vi "Test UI.vi"() -> ()   [LabVIEW 2012]
uses:
  Controls/Settings.ctl
  Controls/Stop.ctl
  Controls/Altitude Xctl/Altitude2.xctl
panel:
  out "Altitude2":cluster{"time":timestamp, "altitude":dbl}(xcontrol)
  in  "Stop":T1
  in  "settings":T2
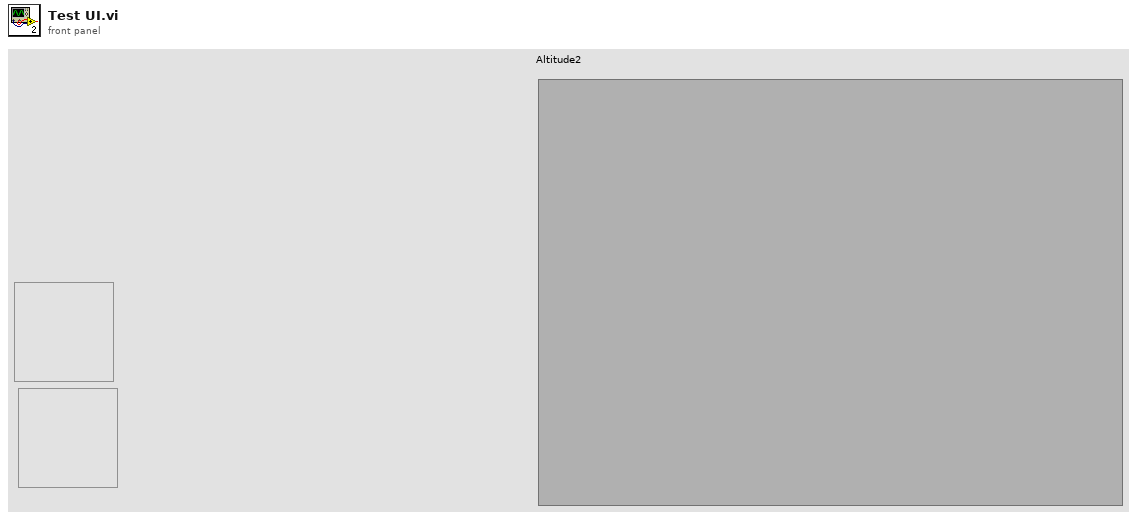
[diagram p1: front panel]
types:
  T1 = typedef "Stop.ctl" = bool
  T2 = typedef "Settings.ctl" = bool
  T3 = cluster{"seconds since 1Jan1904":timestamp, "number: 0 to 1":dbl}
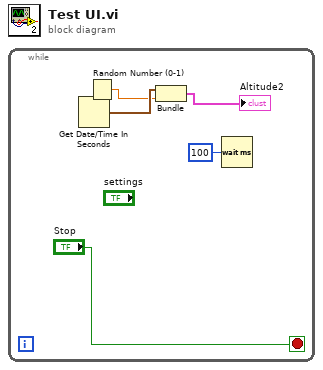
[diagram p0: block diagram]
diagram:
  n1 = while {
    stop <- "Stop" stop-if-true
    n2 = Get Date/Time In Seconds() -> (seconds since 1Jan1904=w3:timestamp)
    n3 = Random Number (0-1)() -> (number: 0 to 1=w2:dbl)
    n4 = Bundle("seconds since 1Jan1904"=w3, "number: 0 to 1"=w2) -> (→"Altitude2":T3)  [unwired: 1 in]
    n5 = Wait (ms)(milliseconds to wait=u32 100) -> ()  [unwired: 1 out]
  }
